vi "make_lut.vi"() -> ()   [LabVIEW 2012]
uses:
  geometry/lut4d.ctl
panel:
  in  "Random probes":i32=100000
  in  "Use range":sgl[](array[numeric])=[0.8, 0.8, 0.8, 0.15]
  out "Test results":T1 {"Max error axis positions" format="%#.4f"; "RMS error" format="%#.1f"; "Max error" format="%#.1f"}
  in  "Output file":path=path "C:/Users/ram/Documents/work/Micron/asap/cal_data/SN1/stage_new/asap_lut.bin"
  out "Result":T2={"Table"=array41x41x41x5x4[1378420 elements], "Scale"=[2.0, 2.0, 2.0, 0.11], "Offset"=[-1.0, -1.0, -1.0, -0.03]}
  in  "Max values":sgl[](array[numeric])=[1.0, 1.0, 1.0, 0.2]
  in  "Min values":sgl[](array[numeric])=[-1.0, -1.0, -1.0, -0.2]
  in  "Interpolate points":i32[](array[numeric])=[41, 41, 41, 7]
  in  "Calibration file name":path=path "C:/Users/ram/Documents/work/Micron/asap/cal_data/SN1/stage_new/calibration.dat"
  # "Error estimate in microns over central part of range.  See test_lut.vi"
  # "Warning:\nThe LUT code assumes the second and 4'th axes (1 and 3) are redundant Z axes.  If for some reason (e.g. sensor orientation) this is not the case we will end up tabulating a useless part of the intersection space. When testing the result, we include only points that have an acceptable Z mismatch, so a sanity check is that \"Points tested\" ends up about 1/10 of \"Random probes\" (rather than zero or nearly so.)\n\nThe  Z mismatch will vary depending on the hardware, can can be gleaned from the calibration results, e.g. measured(:,2)-measured(:,4).   Another sanity check is that the result the match error should cross zero approximately in the middle of the 4'th dimension, i.e. in the vertical center of the 4'th column in the display above.    If we've set the min/max values on the 4'th dimension right, then this should defintely be true at the center of the workspace, at approx (20,20,20), and there should be a zero crossing in the last column except near corners of the table (not corresponding to usable range.)"
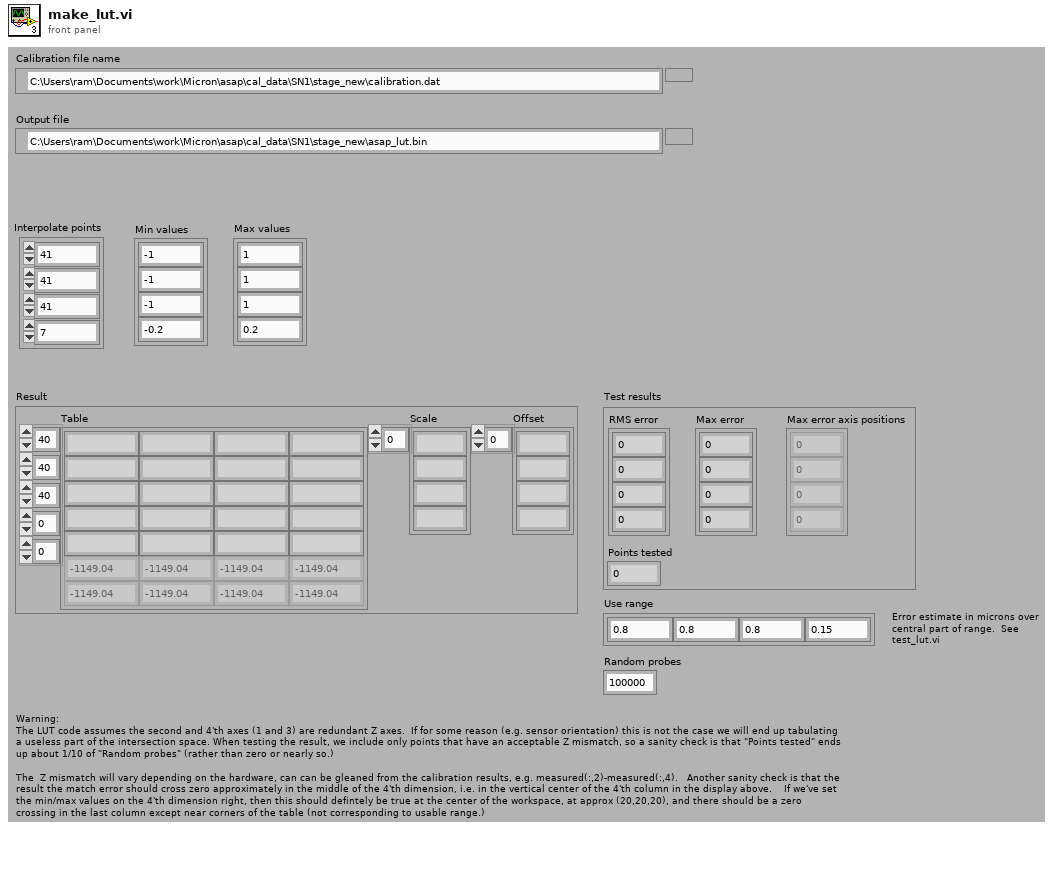
[diagram p1: front panel]
types:
  T1 = cluster{"Max error":sgl[], "Points tested":i32, "RMS error":sgl[], "Max error axis positions":sgl[]}
  T2 = typedef "lut4d.ctl" = cluster{"Table":sgl[][][][][], "Scale":sgl[], "Offset":sgl[]}
  T3 = typedef "asap_calibration.ctl" = cluster{"T1":T4, "K1":T4, "T2":T4, "K2":T4, "Sensor LUT":sgl[][][][]}
  T4 = typedef "NI_Matrix.lvlib/RealMatrix.ctl" = dbl[][]
  T5 = cluster{"Interpolate points[0]":i32, "Interpolate points[1]":i32, "Interpolate points[2]":i32, "Interpolate points[3]":i32}
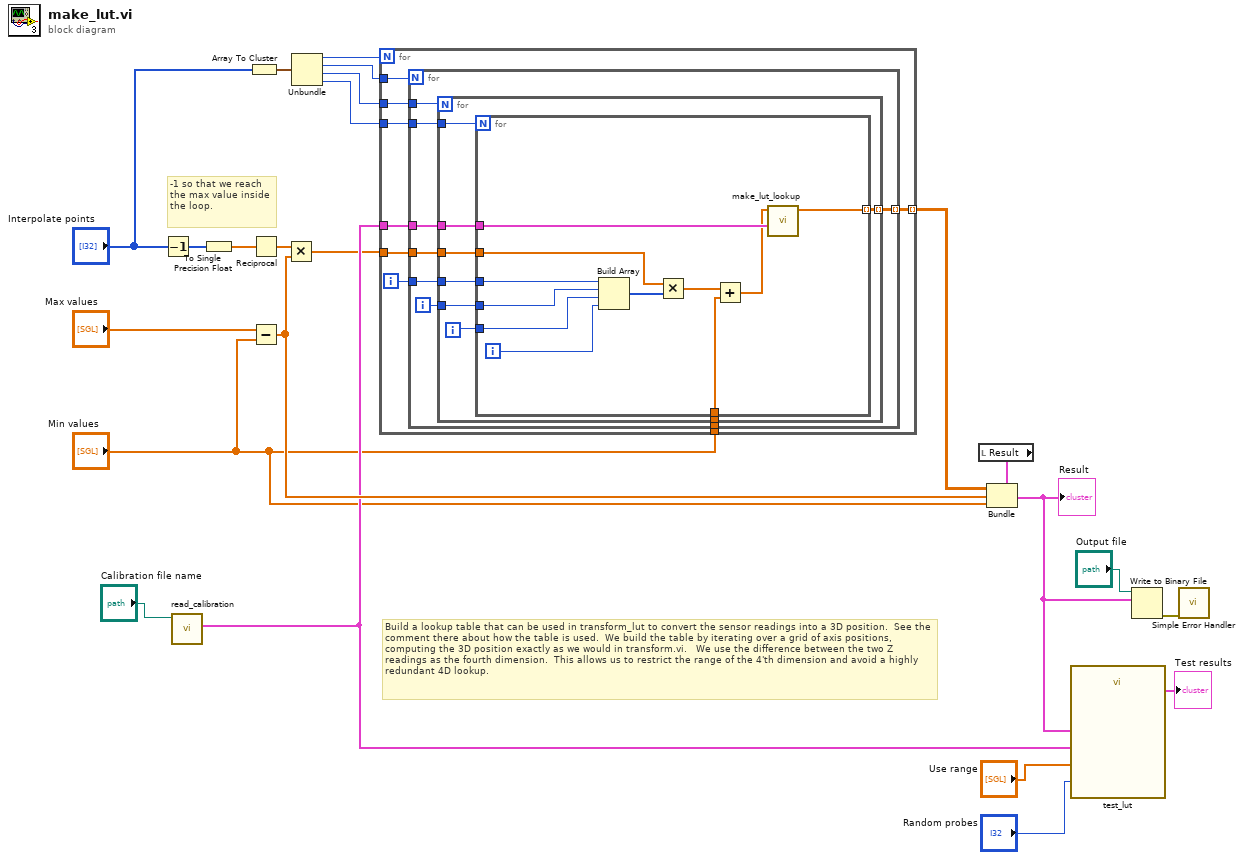
[diagram p0: block diagram]
diagram:
  # "-1 so that we reach the max value inside the loop."
  # "Build a lookup table that can be used in transform_lut to convert the sensor readings into a 3D position.  See the comment there about how the table is used.  We build the table by iterating over a grid of axis positions, computing the 3D position exactly as we would in transform.vi.   We use the difference between the two Z readings as the fourth dimension.  This allows us to restrict the range of the 4'th dimension and avoid a highly redundant 4D lookup."
  n1 = Decrement(x="Interpolate points") -> (x-1=w4:i32[])
  n2 = call "read_calibration.vi"("Calibration file name"="Calibration file name") -> ("Calibration data"=w9:T3)  [unwired: 1 in, 9 out]
  n3 = To Single Precision Float(number=w4) -> (single precision float=w23:sgl[])
  n4 = Array To Cluster(array="Interpolate points") -> (cluster=w21:T5)
  n5 = Reciprocal(x=w23) -> (1/x=w15:sgl[])
  n6 = Subtract(x="Max values", y="Min values") -> (x-y=w13:sgl[])
  n7 = Multiply(x=w15, y=w13) -> (x*y=w6:sgl[])
  n8 = Unbundle(w21) -> ("Interpolate points[0]"=w20:i32, "Interpolate points[1]"=w19:i32, "Interpolate points[2]"=w18:i32, "Interpolate points[3]"=w17:i32)
  n9 = for {
    N: w20 -> [_]
    tunnel: w6 -> [w30]
    tunnel: [w29] -> w14 mode=indexing
    tunnel: w19 -> [w28]
    tunnel: w18 -> [w27]
    tunnel: w17 -> [w26]
    tunnel: "Min values" -> [w25]
    tunnel: w9 -> [w24]
    i -> [w31]
    n10 = for {
      N: w28 -> [_]
      tunnel: w31 -> [w39]
      tunnel: w30 -> [w37]
      tunnel: [w36] -> w29 mode=indexing
      tunnel: w27 -> [w35]
      tunnel: w26 -> [w34]
      tunnel: w25 -> [w33]
      tunnel: w24 -> [w32]
      i -> [w38]
      n11 = for {
        N: w35 -> [_]
        tunnel: w39 -> [w46]
        tunnel: w38 -> [w45]
        tunnel: w37 -> [w47]
        tunnel: [w43] -> w36 mode=indexing
        tunnel: w34 -> [w42]
        tunnel: w33 -> [w41]
        tunnel: w32 -> [w40]
        i -> [w44]
        n12 = for {
          N: w42 -> [_]
          tunnel: w47 -> [w58]
          tunnel: w46 -> [w48]
          tunnel: w45 -> [w49]
          tunnel: w44 -> [w50]
          tunnel: [w57] -> w43 mode=indexing
          tunnel: w41 -> [w54]
          tunnel: w40 -> [w53]
          i -> [w51]
          n13 = Build Array(w48, w49, w50, w51) -> (w56:i32[])
          n14 = Multiply(x=w58, y=w56) -> (x*y=w55:sgl[])
          n15 = Add(x=w55, y=w54) -> (x+y=w52:sgl[])
          n16 = call "make_lut_lookup.vi"("Calibration data"=w53, "LUT inputs"=w52) -> ("XYZ and match error"=w57:sgl[])  [unwired: 8 in, 1 out]
        }
      }
    }
  }
  n17 = local read "Result"() -> (w12:T2)
  n18 = Bundle(cluster=w12, "Table"=w14, "Scale"=w13, "Offset"="Min values") -> (w8:T2)
  "Result" <- w8
  n19 = call "test_lut.vi"("Use range"="Use range", "Random probes"="Random probes", "Calibration data"=w9, "LUT"=w8) -> ("Results"=→"Test results":T1)  [unwired: 7 in]
  n20 = Write to Binary File(file (use dialog)="Output file", data=w8) -> (error out=w10:errorcluster)  [unwired: 1 in, 5 out]
  n21 = call <vilib>:"Simple Error Handler.vi"("error in (no error)"=w10) -> ()  [unwired: 1 in, 8 out]
